vi "FleaAbsorptionImaging.vi"() -> ()   [LabVIEW 2013] (continued)
  in  "Save files to archive?":bool
  out "Timeout":bool=TRUE
  out "Trigger Overrun":bool=TRUE
  in  "Source of File Data":refnum<k21>="\\\\localhost\\VariableLibrary\\Instruction String"
  in  "Timeout (ms)":u32=20000
  in  "Gain":dbl
  in  "Shutter speed (ms)":dbl=0.15
  in  "Source of Wavemeter Data":refnum<k21>="\\\\WS7PC\\VariableLibrary\\Frequency"
  in  "Accept wavelength from remote system":bool
  in  "Flea Raw image to view":u16(ring) items=["Absorbtion", "Probe", "Background"]
  in  "Update Graphics":bool=TRUE
  out "Flea Raw Image":u16[][](graph)
  out "Flea Processed Image":sgl[][](graph)
  out "Camera Error":errorcluster={"status"=FALSE, "code"=-1074360293, "source"="IMAQdx Get Image.vi"}
  out "Status Array":T4(array[cluster])=[{"AcquisitionInProgress"=FALSE, "BufferCount"=1164, "LastBufferNumber"=1163, "LostBufferCount"=0}, {"AcquisitionInProgress"=TRUE, "BufferCount"=12297, "LastBufferNumber"=12296, "LostBufferCount"=0}, {"AcquisitionInProgress"=TRUE, "BufferCount"=12298, "LastBufferNumber"=12297, "LostBufferCount"=0}, {"AcquisitionInProgress"=TRUE, "BufferCount"=12299, "LastBufferNumber"=12298, "LostBufferCount"=0}, {"AcquisitionInProgress"=TRUE, "BufferCount"=12300, "LastBufferNumber"=12299, "LostBufferCount"=0}]
  out "Flea Images":u16[][][](array[numeric])
  out "Buffer Number":u32=4294967294
  out "Flea Frames":i32
  out "Flea Loop":i32=3073
  # "Image Acquisition v4.5"
  # "Experimental Parameters"
  # "These are only get set on 1st run.\nUse a Gain of 0, Shutter Speed not used"
  # "In both techniques 3 images\nare aquired, but in Fluorescense\nthe 3rd is discarded"
  # "Sr: .663  is XZ a\n     .898 is XZ b\n      5.48 is XY"
  # "Obsolete: (now done with network variables)\nWhen paramaters are accepted from a remote system a DataSockets server\nmust be running on this machine (in start menu in National Instruments folder)"
  # "Camera configuration"
  # "File configuration"
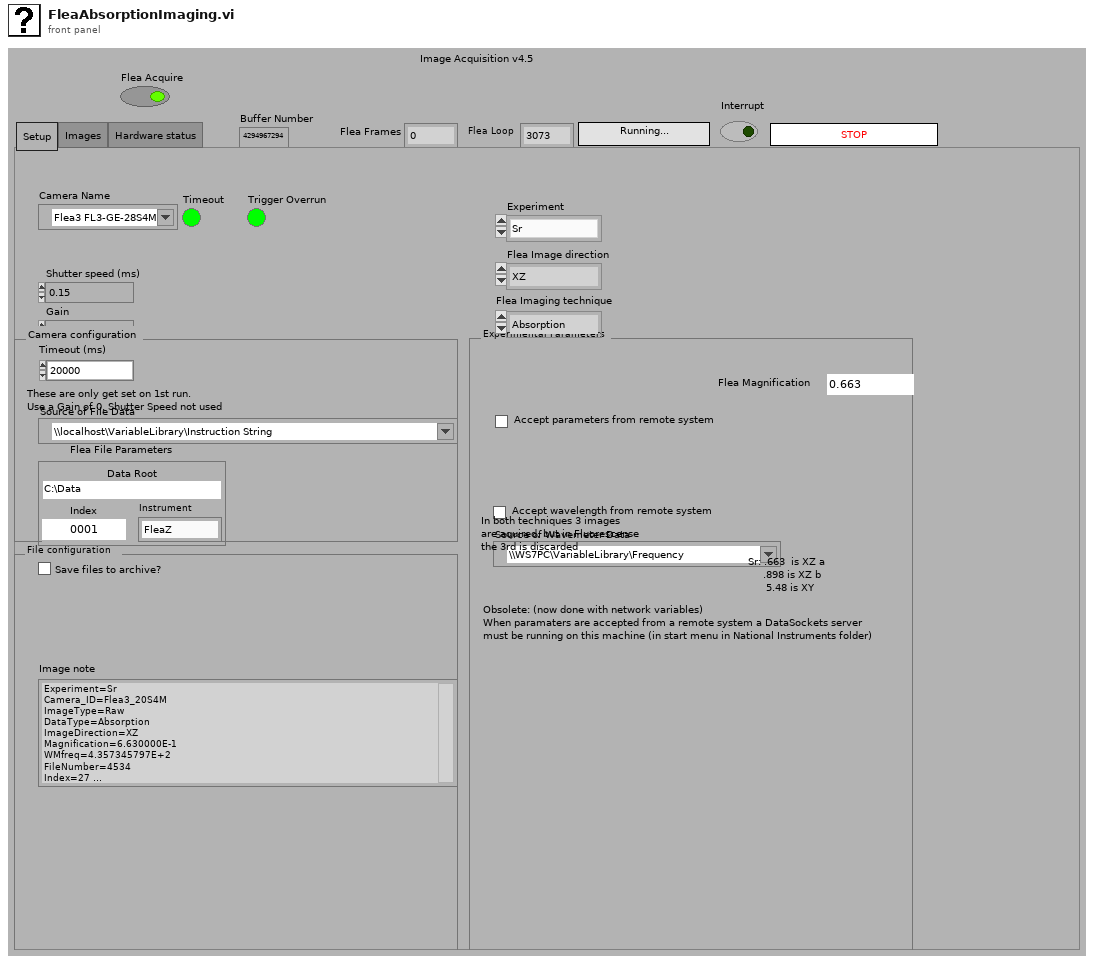
[diagram p1: front panel]
types:
  T1 = typedef "FileName_Cluster.ctl" = cluster{"Data Root":path, "Index":u32, "Instrument":string}
  T2 = typedef "IMAQdx.ctl" = refnum<k21>
  T3 = enum16{"Rubidium I", "Rubidium II", "RbLi", "RbYb", "Sr"}
  T4 = cluster{"AcquisitionInProgress":bool, "BufferCount":u32, "LastBufferNumber":u32, "LostBufferCount":u32}[]
  T5 = typedef "NI_Vision_Acquisition_Software.lvlib/IMAQdx Acquisition Mode.ctl" = enum32{"One Shot", "Continuous"}
  T6 = typedef "H5F.lvlib/H5Fmode.ctl" = enum16{"read-only", "read-write", "overwrite", "create new", "open or create"}
  T7 = typedef "Image Type" = u32
  T8 = typedef "IMAQ Image.ctl" = refnum<image>
  T9 = cluster{"AcquisitionInProgress":bool, "BufferCount":u32, "LastBufferNumber":u32, "LostBufferCount":u32}
  T10 = typedef "hid_t.ctl" = i32
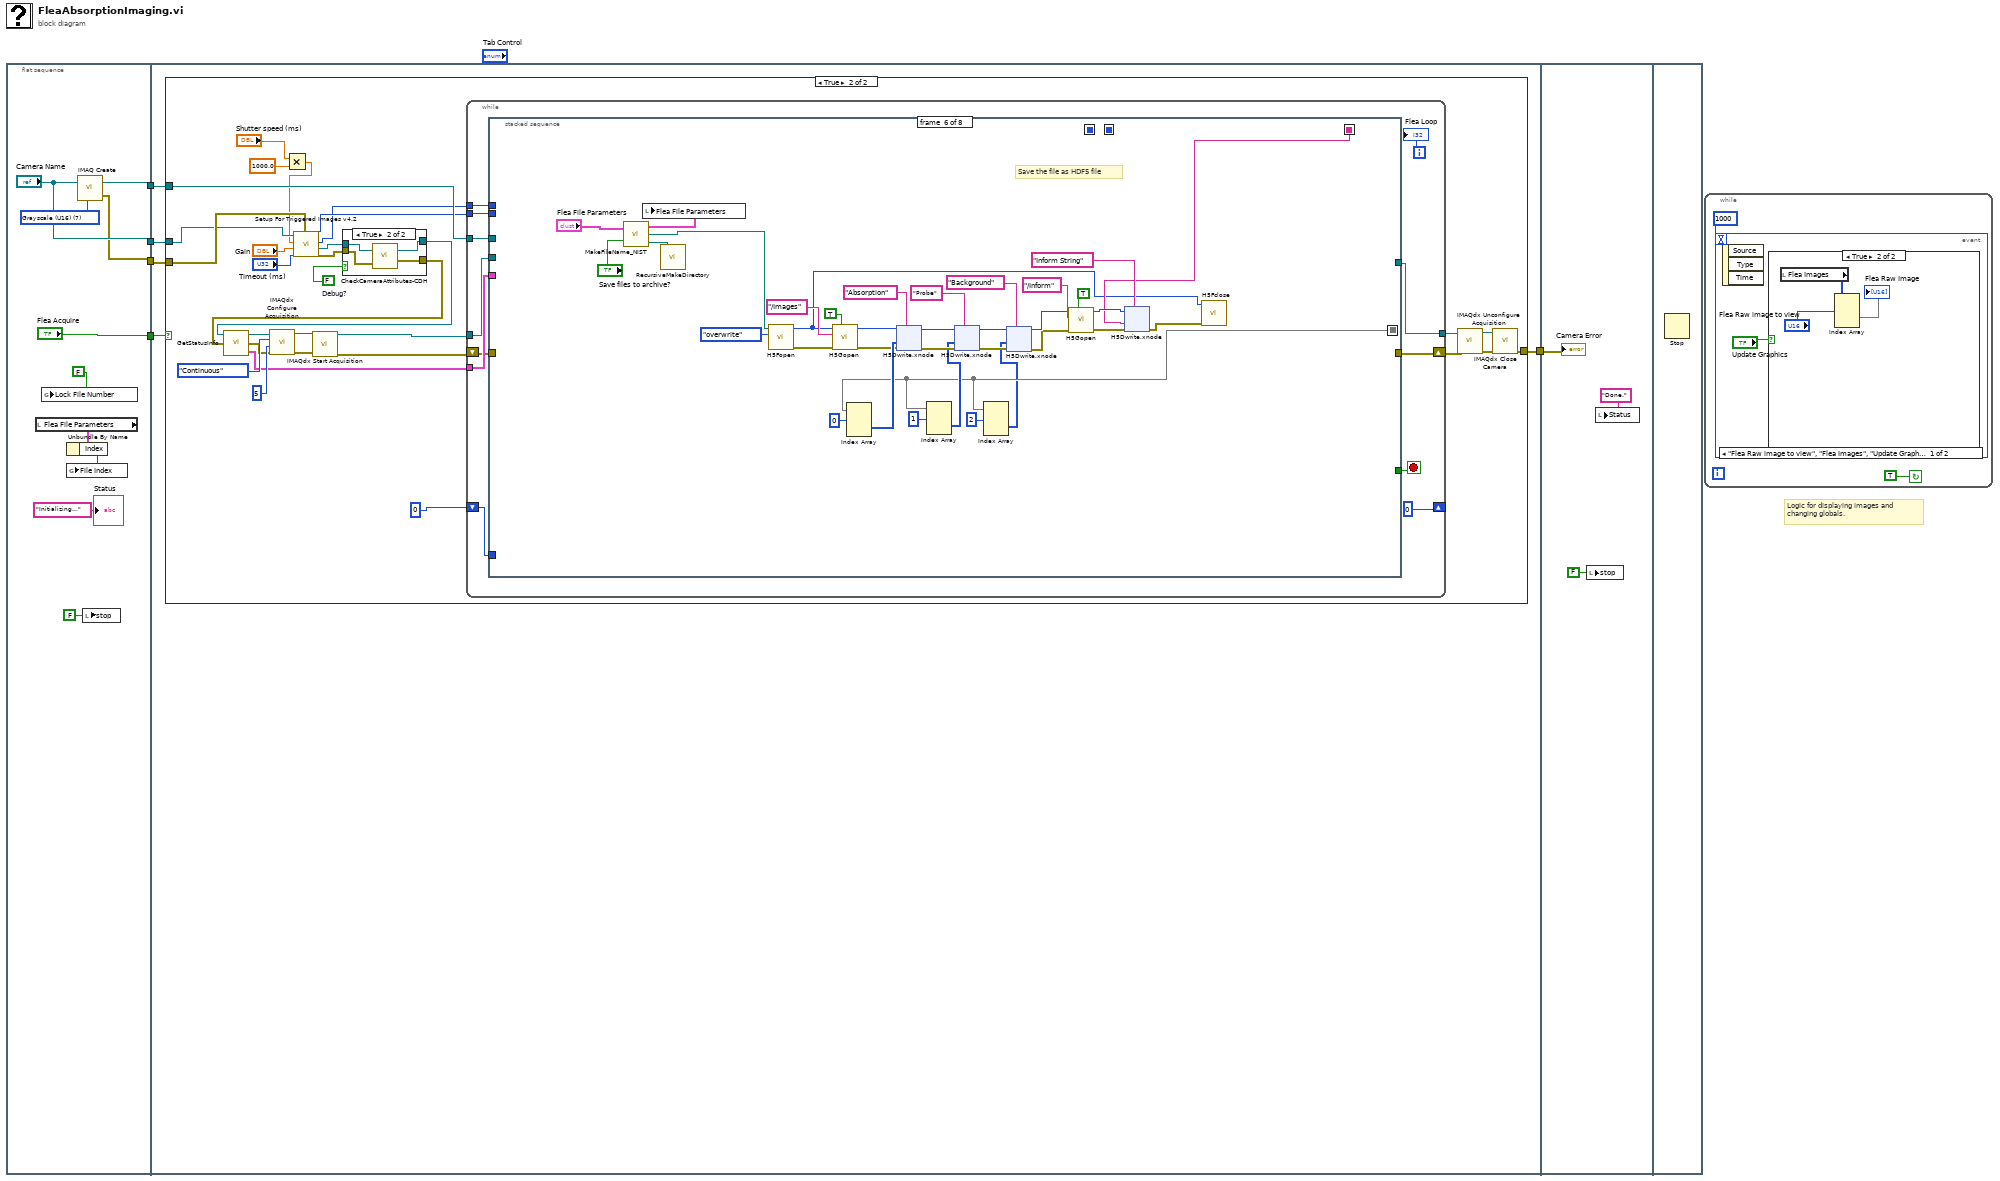
[diagram p0: block diagram]
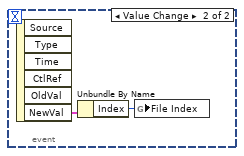
[diagram p3: hidden frame]
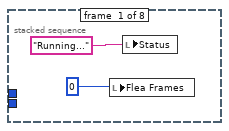
[diagram p6: hidden frame]
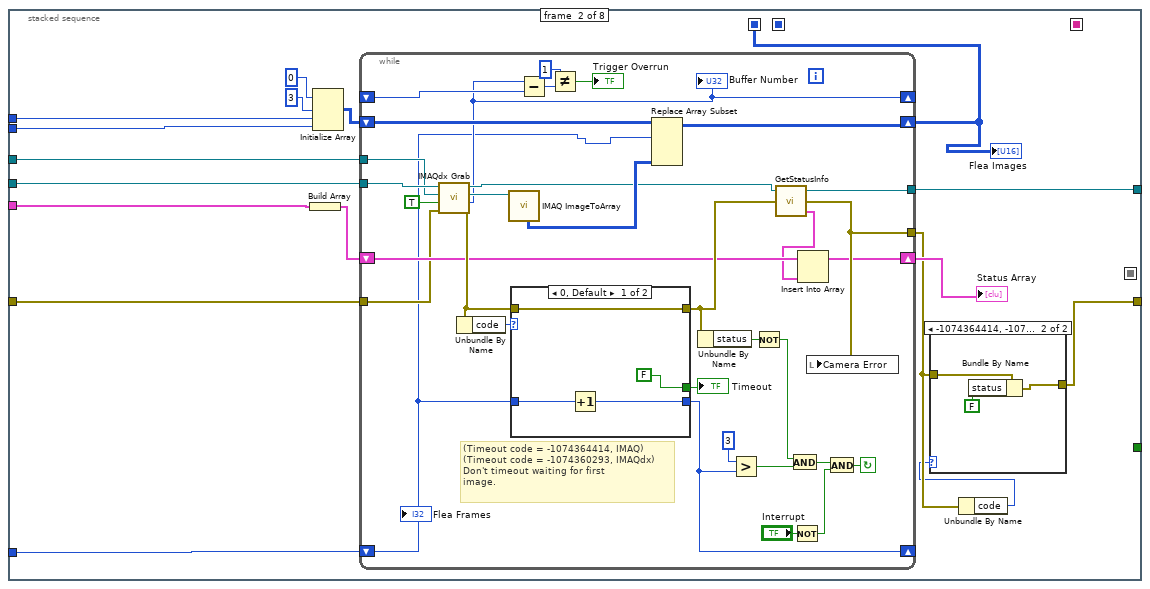
[diagram p7: hidden frame]
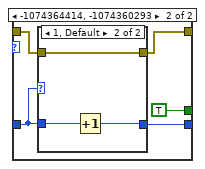
[diagram p9: hidden frame]
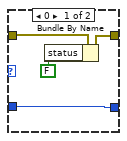
[diagram p10: hidden frame]
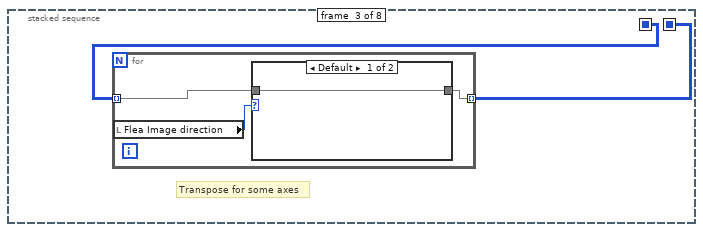
[diagram p11: hidden frame]
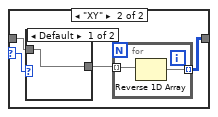
[diagram p12: hidden frame]
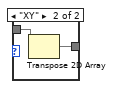
[diagram p13: hidden frame]
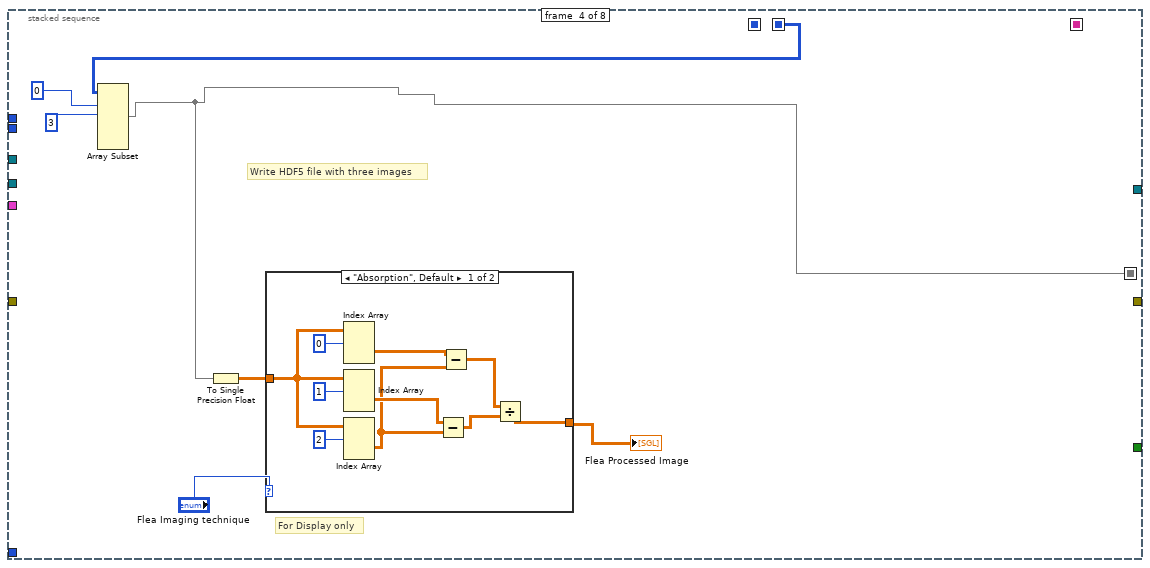
[diagram p14: hidden frame]
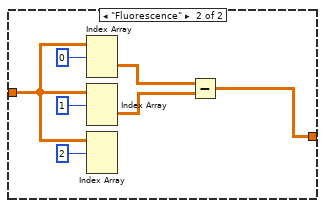
[diagram p15: hidden frame]
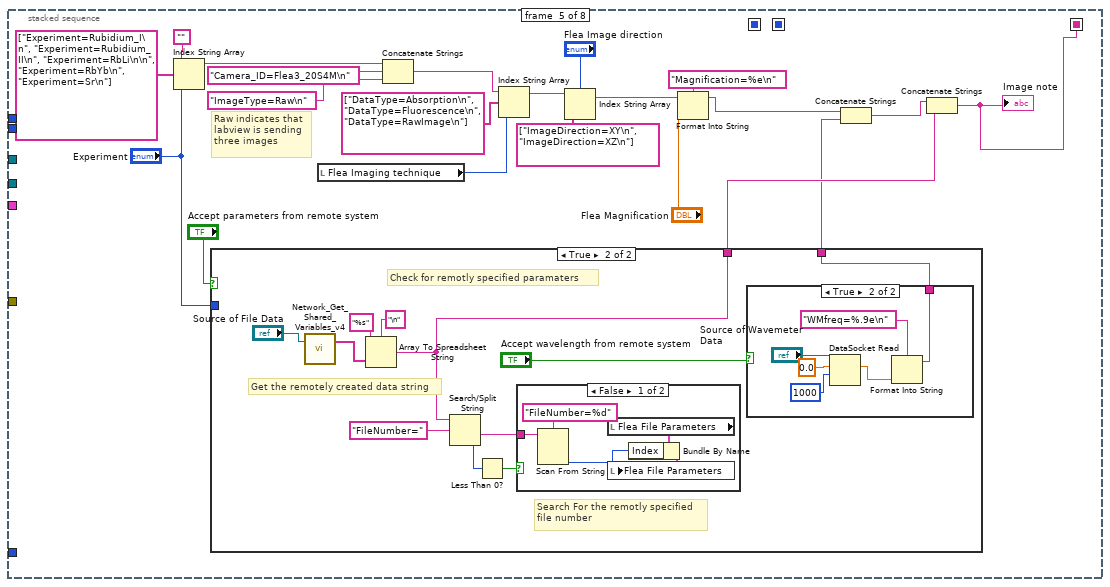
[diagram p16: hidden frame]
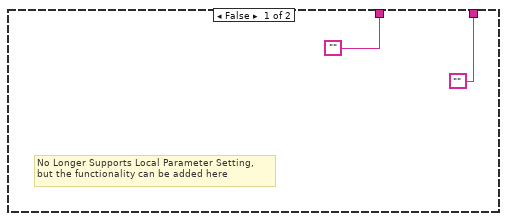
[diagram p17: hidden frame]
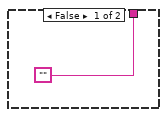
[diagram p18: hidden frame]
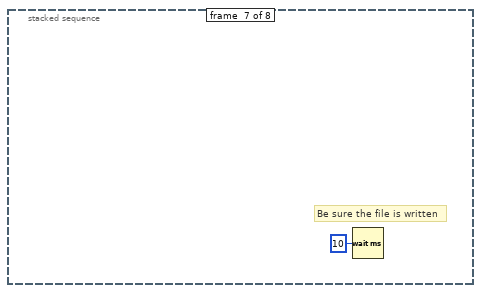
[diagram p20: hidden frame]
diagram:
  # "Logic for displaying images and\nchanging globals."
  n1 = flat-sequence {
    tunnel: [w11] -> w5
    tunnel: ["Camera Name"] -> w4
    tunnel: [w9] -> w3
    tunnel: ["Flea Acquire"] -> w1
    tunnel: w4 -> [w20]
    tunnel: w5 -> [w18]
    tunnel: w3 -> [w19]
    tunnel: [w17] -> w2
    tunnel: w1 -> [w16]
    tunnel: w2 -> [w337]
    frame #0 {
      w8 = T7 7 items=["Grayscale (U8)", "Grayscale (I16)", "Grayscale (SGL)", "Complex (CSG)", "RGB (U32)", "HSL (U32)", "RGB (U64)", "Grayscale (U16)"] ("Image Type")
      n2 = local read "Flea File Parameters"() -> (w12:T1)
      n3 = global write "FileInfo_Global.vi" "Lock File Number"(FALSE) -> ()
      n4 = Unbundle By Name(w12) -> ("Index"=w13:u32)
      n5 = global write "FileInfo_Global.vi" "File Index"(w13) -> ()
      n6 = call "IMAQ Create"("Image Name"="Camera Name", "Image Type"=w8) -> ("New Image"=w11:T8, "error out"=w9:errorcluster)  [unwired: 2 in, 1 out]
      n7 = local write "stop"(FALSE ("stop")) -> ()
      "Status" <- "Initializing..."
    }
    frame #1 {
      n8 = case shown="True" w16 {
        tunnel: w20 -> [_ w27]
        tunnel: w19 -> [w21 w28]
        tunnel: w18 -> [_ w41]
        tunnel: [w21 w35] -> w17
        frame False {
        }
        frame True {
          w49 = FALSE  # Debug?
          n9 = Multiply(x="Shutter speed (ms)", y=1000.0) -> (x*y=w22:dbl)
          n10 = call "Setup For Triggered Images v4.2.vi"("error in"=w28, "Timeout (ms)"="Timeout (ms)", "Gain"="Gain", "Shutter Speed (us)"=w22, "Camera Name"=w27) -> ("Error out"=w29:errorcluster, "Session Out"=w30:T2, "Height"=w31:u32, "Width"=w32:u32)
          n11 = case shown="True" w49 {
            tunnel: [w52 w57] -> w48
            tunnel: [w53 w56] -> w45
            tunnel: w30 -> [w52 w55]
            tunnel: w29 -> [w53 w54]
            frame False {
            }
            frame True {
              n12 = call "CheckCameraAttributes-CDH.vi"("error in"=w54, "Camera Name"=w55) -> ("error out"=w56:errorcluster, "Session Out"=w57:T2)
            }
          }
          n13 = call "GetStatusInfo.vi"("error in"=w45, "Camera In"=w48) -> ("Status Info"=w40:T9, "error out"=w46:errorcluster, "Camera Out"=w47:T2)  [unwired: 1 in]
          n14 = call <vilib>:"IMAQdx Configure Acquisition.vi"("error in"=w46, "Number of Buffers"=u32 5, "Continuous?"=IMAQdx_Acquisition_Mode."Continuous", "Session In"=w47) -> ("error out"=w43:errorcluster, "Session Out"=w44:T2)  [unwired: 6 in]
          n15 = call <vilib>:"IMAQdx Start Acquisition.vi"("error in"=w43, "Session In"=w44) -> ("error out"=w38:errorcluster, "Session Out"=w42:T2)  [unwired: 8 out]
          n16 = while {
            tunnel: w42 -> [w67]
            tunnel: w41 -> [w66]
            tunnel: w31 -> [w65]
            tunnel: w32 -> [w64]
            tunnel: w40 -> [w63]
            tunnel: [w62] -> w34
            shift-right: [0] -> _
            shift-left: 0 -> [w61]
            shift-right: [w58] -> w37
            shift-left: w38 -> [w59]
            i -> [w69]
            stop <- w68 stop-if-true
            n17 = stacked-sequence {
              seq-local: [_ _ _ w157 _ _ _ _] -> [_ _ _ _ _ w240 _ _]
              seq-local: [_ w72 _ _ _ _ _ _] -> [_ _ w143 _ _ _ _ _]
              seq-local: [_ _ w142 _ _ _ _ _] -> [_ _ _ w160 _ _ _ _]
              seq-local: [_ _ _ _ w181 _ _ _] -> [_ _ _ _ _ w229 _ _]
              tunnel: [_ _ _ _ _ _ _ "stop"] -> w68
              tunnel: w67 -> [_ w84 _ _ _ _ _ _]
              tunnel: w66 -> [_ w83 _ _ _ _ _ _]
              tunnel: w65 -> [_ w82 _ _ _ _ _ _]
              tunnel: w64 -> [_ w81 _ _ _ _ _ _]
              tunnel: w63 -> [_ w79 _ _ _ _ _ _]
              tunnel: [_ w78 _ _ _ _ _ _] -> w62
              tunnel: [_ w75 _ _ _ _ _ _] -> w58
              tunnel: w61 -> [_ w77 _ _ _ _ _ _]
              tunnel: w59 -> [_ w76 _ _ _ _ _ _]
              frame #0 {
                n18 = local write "Flea Frames"(0) -> ()
                n19 = local write "Status"("Running...") -> ()
              }
              frame #1 {
                n20 = Build Array(w79) -> (w80:T4)
                n21 = Initialize Array(u16 0, 3, w82, w81) -> (w86:u16[][][])
                n22 = while {
                  shift-right: [w97] -> _
                  shift-left: _ -> [w120]
                  tunnel: [w104] -> w78
                  tunnel: [w101] -> w74
                  shift-right: [w111] -> _
                  shift-left: w77 -> [w93]
                  shift-right: [w116] -> w72
                  shift-left: w86 -> [w117]
                  shift-right: [w99] -> w85
                  shift-left: w80 -> [w100]
                  tunnel: w84 -> [w96]
                  tunnel: w83 -> [w95]
                  tunnel: w76 -> [w94]
                  stop <- w107 continue-if-true
                  # "(Timeout code = -1074364414, IMAQ)\n(Timeout code = -1074360293, IMAQdx)\nDon't timeout waiting for first\nimage."
                  n23 = call <vilib>:"IMAQdx Grab.vi"("error in"=w94, "Wait for Next Buffer? (Yes)"=TRUE, "Image In"=w95, "Session In"=w96) -> ("error out"=w115:errorcluster, "Buffer Number Out"=w97:u32, "Image Out"=w110:T8, "Session Out"=w103:T2)  [unwired: 4 out]
                  "Buffer Number" <- w97
                  n24 = Unbundle By Name(w115) -> ("code"=w124:i32)
                  n25 = call "IMAQ ImageToArray"("Image"=w110) -> ("Image Pixels (U16)"=w109:u16[][])  [unwired: 2 in, 5 out]
                  n26 = case shown="0, Default" w124 {
                    tunnel: w115 -> [w129 w133]
                    tunnel: [w129 w132] -> w102
                    tunnel: [FALSE TRUE] -> w125
                    tunnel: w93 -> [w127 w131]
                    tunnel: [w126 w130] -> w111
                    frame 0, Default {
                      n27 = Increment(x=w127) -> (x+1=w126:i32)
                    }
                    frame -1074364414, -1074360293 {
                      n28 = case shown="1, Default" w131 {
                        tunnel: [w135 w141] -> w132
                        tunnel: w133 -> [w137 w141]
                        tunnel: w131 -> [w136 w140]
                        tunnel: [w136 w139] -> w130
                        frame 0 {
                          n29 = Bundle By Name(cluster=w137, "status"=FALSE) -> (w135:errorcluster)
                        }
                        frame 1, Default {
                          n30 = Increment(x=w140) -> (x+1=w139:i32)
                        }
                      }
                    }
                  }
                  "Timeout" <- w125
                  n31 = Subtract(x=w97, y=w120) -> (x-y=w121:u32)
                  n32 = Not Equal?(x=u32 1, y=w121) -> (x != y?=→"Trigger Overrun":bool)
                  n33 = Replace Array Subset(array=w117, new element=w109, index (dim 0)=w93) -> (w116:u16[][][])  [unwired: 2 in]
                  n34 = Unbundle By Name(w102) -> ("status"=w119:bool)
                  n35 = Greater?(x=3, y=w111) -> (0:w112:bool)
                  n36 = Not(x=w119) -> (.not. x?=w118:bool)
                  n37 = call "GetStatusInfo.vi"("error in"=w102, "Camera In"=w103) -> ("Status Info"=w98:T9, "error out"=w101:errorcluster, "Camera Out"=w104:T2)  [unwired: 1 in]
                  n38 = And(x=w118, y=w112) -> (x .and. y?=w108:bool)
                  n39 = Not(x="Interrupt") -> (.not. x?=w105:bool)
                  n40 = Insert Into Array(array=w100, new element=w98) -> (w99:T4)  [unwired: 1 in]
                  n41 = local write "Camera Error"(w101) -> ()
                  n42 = And(x=w108, y=w105) -> (x .and. y?=w107:bool)
                  "Flea Frames" <- w93
                }
                "Flea Images" <- w72
                "Status Array" <- w85
                n43 = Unbundle By Name(w74) -> ("code"=w73:i32)
                n44 = case shown="-1074364414, -1074360293" w73 {
                  tunnel: [w89 w91] -> w75
                  tunnel: w74 -> [w89 w90]
                  frame 0, Default {
                  }
                  frame -1074364414, -1074360293 {
                    n45 = Bundle By Name(cluster=w90, "status"=FALSE) -> (w91:errorcluster)
                  }
                }
              }
              frame #2 {
                # "Transpose for some axes"
                n46 = for {
                  tunnel: w143 -> [w145] mode=indexing
                  tunnel: [w144] -> w142 mode=indexing
                  n47 = local read "Flea Image direction"() -> (w146:enum16{"XY", "XZ"})
                  n48 = case shown="Default" w146 {
                    selector: w146 -> [_ w148]
                    tunnel: w145 -> [w147 w150]
                    tunnel: [w147 w151] -> w144
                    frame Default {
                    }
                    frame "XY" {
                      n49 = case shown="Default" w148 {
                        tunnel: w150 -> [w152 w154]
                        tunnel: [w152 w153] -> w149
                        frame Default {
                        }
                        frame "XY" {
                          n50 = Transpose 2D Array(2D array=w154) -> (transposed array=w153:u16[][])
                        }
                      }
                      n51 = for {
                        tunnel: w149 -> [w156] mode=indexing
                        tunnel: [w155] -> w151 mode=indexing
                        n52 = Reverse 1D Array(array=w156) -> (reversed array=w155:u16[])
                      }
                    }
                  }
                }
              }
              frame #3 {
                # "Write HDF5 file with three images"
                # "For Display only"
                n53 = Array Subset(array=w160, index (dim 0)=0 ("index"), length (dim 0)=3 ("length")) -> (w157:u16[][][])  [unwired: 4 in]
                n54 = To Single Precision Float(number=w157) -> (single precision float=w161:sgl[][][])
                n55 = case shown="\"Absorption\", Default" "Flea Imaging technique" {
                  tunnel: [w170 w176] -> w162
                  tunnel: w161 -> [w169 w177]
                  frame "Absorption", Default {
                    n56 = Index Array(array=w169, index (dim 0)=0 ("Number of buffers")) -> (element=w168:sgl[][])  [unwired: 2 in]
                    n57 = Index Array(array=w169, index (dim 0)=1 ("Number of buffers")) -> (element=w167:sgl[][])  [unwired: 2 in]
                    n58 = Index Array(array=w169, index (dim 0)=2 ("Number of buffers")) -> (element=w166:sgl[][])  [unwired: 2 in]
                    n59 = Subtract(x=w167, y=w166) -> (x-y=w165:sgl[][])
                    n60 = Subtract(x=w168, y=w166) -> (x-y=w164:sgl[][])
                    n61 = Divide(x=w164, y=w165) -> (x/y=w170:sgl[][])
                  }
                  frame "Fluorescence" {
                    n62 = Index Array(array=w177, index (dim 0)=0 ("Number of buffers")) -> (element=w175:sgl[][])  [unwired: 2 in]
                    n63 = Index Array(array=w177, index (dim 0)=1 ("Number of buffers")) -> (element=w174:sgl[][])  [unwired: 2 in]
                    n64 = Index Array(array=w177, index (dim 0)=2 ("Number of buffers")) -> ()  [unwired: 2 in, 1 out]
                    n65 = Subtract(x=w175, y=w174) -> (x-y=w176:sgl[][])
                  }
                }
                "Flea Processed Image" <- w162
              }
              frame #4 {
                # "Raw indicates that\nlabview is sending\nthree images"
                n66 = Index String Array(1:"Experiment", 2:string[] ["Experiment=Rubidium_I\n", "Experiment=Rubidium_II\n", "Experiment=RbLi\n\n", "Experiment=RbYb\n", "Experiment=Sr\n"], 3:"") -> (0:w189:string)
                n67 = case shown="True" "Accept parameters from remote system" {
                  tunnel: ["" w207] -> w194
                  tunnel: "Experiment" -> [_ _]
                  tunnel: ["" w204] -> w182
                  frame False {
                    # "No Longer Supports Local Parameter Setting,\nbut the functionality can be added here"
                  }
                  frame True {
                    # "Check for remotly specified paramaters"
                    # "Get the remotely created data string"
                    # "Search For the remotly specified\nfile number"
                    n68 = call "Network_Get_Shared_Variables_v4.vi"("Source of Data"="Source of File Data") -> ("Igor Instruction String"=w214:string[])  [unwired: 1 in, 1 out]
                    n69 = Array To Spreadsheet String(delimiter (Tab)="\n", array=w214, 3:"%s") -> (spreadsheet string=w207:string)
                    n70 = Search/Split String(string=w207, search string/char (-)="FileNumber=") -> (match + rest of string=w210:string, offset of match=w209:i32)  [unwired: 2 out]
                    n71 = Less Than 0?(x=w209) -> (x < 0?=w208:bool)
                    n72 = case shown="False" w208 {
                      tunnel: w210 -> [w226 _]
                      frame False {
                        n73 = Scan From String(format string="FileNumber=%d", input string=w226) -> (output 1=w222:i32)  [unwired: 2 in, 4 out]
                        n74 = local read "Flea File Parameters"() -> (w224:T1)
                        n75 = Bundle By Name(cluster=w224, "Index"=w222) -> (w223:T1)
                        n76 = local write "Flea File Parameters"(w223) -> ()
                      }
                      frame True {
                      }
                    }
                    n77 = case shown="True" "Accept wavelength from remote system" {
                      tunnel: ["" w216] -> w204
                      frame False {
                      }
                      frame True {
                        n78 = DataSocket Read(9:1000 ("ms timeout (10000)"), 10:0.0, 11:"Source of Wavemeter Data") -> (2:w219:dbl)  [unwired: 2 in, 6 out]
                        n79 = Format Into String(format string="WMfreq=%.9e\n", w219) -> (resulting string=w216:string)  [unwired: 2 in, 1 out]
                      }
                    }
                  }
                }
                n80 = local read "Flea Imaging technique"() -> (w198:enum16{"Absorption", "Fluorescence", "RawImage"})
                n81 = Concatenate Strings(w189, "Camera_ID=Flea3_20S4M\n", "ImageType=Raw\n") -> (w190:string)
                n82 = Index String Array(1:w198, 2:string[] ["DataType=Absorption\n", "DataType=Fluorescence\n", "DataType=RawImage\n"], 3:w190) -> (0:w199:string)
                n83 = Index String Array(1:"Flea Image direction", 2:string[] ["ImageDirection=XY\n", "ImageDirection=XZ\n"], 3:w199) -> (0:w201:string)
                n84 = Format Into String(format string="Magnification=%e\n", initial string=w201, "Flea Magnification") -> (resulting string=w183:string)  [unwired: 1 in, 1 out]
                n85 = Concatenate Strings(w183, w182) -> (w184:string)
                n86 = Concatenate Strings(w184, w194) -> (w181:string)
                "Image note" <- w181
              }
              frame #5 {
                # "Save the file as HDF5 file"
                n87 = call "MakeFileName_NIST.vi"("File Parameters"="Flea File Parameters", "Save permanent file?"="Save files to archive?") -> ("New file parameters."=w259:T1, "Path to File"=w256:path, "path"=w260:path)
                n88 = local write "Flea File Parameters"(w259) -> ()
                n89 = call "RecursiveMakeDirectory.vi"("Directory to create"=w260) -> ()  [unwired: 1 in, 2 out]
                n90 = call <vilib>:"H5Fopen.vi"("mode (read-only)"=H5Fmode."overwrite", "path"=w256) -> ("error out"=w237:errorcluster, "ref out"=w228:T10)  [unwired: 8 in]
                n91 = call <vilib>:"H5Gopen.vi"("create? (F)"=TRUE, "error in (no error)"=w237, "name"="/Images", "ref in"=w228) -> ("error out"=w249:errorcluster, "group out"=w250:T10)  [unwired: 6 in]
                n92 = Index Array(array=w240, index (dim 0)=0 ("index (page)")) -> (element=w252:u16[][])  [unwired: 2 in]
                n93 = xnode "H5Dwrite.xnode"("dataset name"="Absorption", "error in (no error)"=w249, "data"=w252, "ref in"=w250) -> ("error out"=w247:errorcluster, "ref out"=w248:i32)  [unwired: 3 in, 1 out]
                n94 = Index Array(array=w240, index (dim 0)=1 ("index (page)")) -> (element=w241:u16[][])  [unwired: 2 in]
                n95 = xnode "H5Dwrite.xnode"("dataset name"="Probe", "error in (no error)"=w247, "data"=w241, "ref in"=w248) -> ("error out"=w243:errorcluster, "ref out"=w244:i32)  [unwired: 3 in, 1 out]
                n96 = Index Array(array=w240, index (dim 0)=2 ("index (page)")) -> (element=w239:u16[][])  [unwired: 2 in]
                n97 = xnode "H5Dwrite.xnode"("dataset name"="Background", "error in (no error)"=w243, "data"=w239, "ref in"=w244) -> ("error out"=w233:errorcluster, "ref out"=w234:i32)  [unwired: 3 in, 1 out]
                n98 = call <vilib>:"H5Gopen.vi"("create? (F)"=TRUE, "error in (no error)"=w233, "name"="/Inform", "ref in"=w234) -> ("error out"=w230:errorcluster, "group out"=w232:T10)  [unwired: 6 in]
                n99 = xnode "H5Dwrite.xnode"("dataset name"="Inform String", "error in (no error)"=w230, "data"=w229, "ref in"=w232) -> ("error out"=w227:errorcluster)  [unwired: 3 in, 2 out]
                n100 = call <vilib>:"H5Fclose.vi"("error in (no error)"=w227, "ref"=w228) -> ()  [unwired: 9 in, 1 out]
              }
              frame #6 {
                # "Be sure the file is written"
                n101 = Wait (ms)(milliseconds to wait=u32 10) -> ()  [unwired: 1 out]
              }
              frame #7 {
              }
            }
            "Flea Loop" <- w69
          }
          n102 = call <vilib>:"IMAQdx Unconfigure Acquisition.vi"("error in"=w37, "Session In"=w34) -> ("error out"=w36:errorcluster, "Session Out"=w33:T2)  [unwired: 8 in]
          n103 = call <vilib>:"IMAQdx Close Camera.vi"("error in"=w36, "Session In"=w33) -> ("error out"=w35:errorcluster)  [unwired: 9 out]
        }
      }
    }
    frame #2 {
      n104 = local write "stop"(FALSE ("stop")) -> ()
      n105 = local write "Status"("Done.") -> ()
      "Camera Error" <- w337
    }
    frame #3 {
      n106 = Stop() -> ()  [unwired: 1 out]
    }
  }
  n107 = while {
    stop <- TRUE continue-if-true
    n108 = event shown="[0] \"Flea Raw image to view\", \"Flea Images\", \"Update Graphics\": Value Change;  Timeout" {
      selector: _ -> [_ _]
      dyn-events: _ -> [_ _]
      timeout: 1000 -> [_ _]
      event "Flea Raw image to view", "Flea Images", "Update Graphics": Value Change; Timeout {
        n109 = event-data() -> ()  [unwired: 4 out]
        n110 = case shown="True" "Update Graphics" {
          frame False {
          }
          frame True {
            n111 = local read "Flea Images"() -> (w344:u16[][][])
            n112 = Index Array(array=w344, index (dim 0)="Flea Raw image to view") -> (element=→"Flea Raw Image":u16[][])  [unwired: 2 in]
          }
        }
      }
      event Value Change {
        n113 = event-data() -> ("NewVal"=w345:T1)  [unwired: 6 out]
        n114 = Unbundle By Name(w345) -> ("Index"=w346:u32)
        n115 = global write "FileInfo_Global.vi" "File Index"(w346) -> ()
      }
    }
  }
